vi "Dresden R2R Sputter 03.02.2018 IY24.vi"() -> ()   [LabVIEW 2009] (continued)
                                }
                                }
                                n29134 = local read "Semi"() -> (w34103:bool)
                                n29135 = Or(x=w34104, y=w34103) -> (x .or. y?=w34099:bool)
                                }
                                }
                                frame #4 {
                                n29136 = local read "Semi"() -> (w34113:bool)
                                n29137 = case shown="False" w34113 {
                                frame #0 {
                                n29138 = while {
                                i -> [w34119]
                                stop <- w34116 stop-if-true
                                n29139 = Greater?(x=w34119, y=50) -> (0:w34118:bool)
                                n29140 = case shown="True" w34118 {
                                frame #0 {
                                }
                                frame #1 {
                                n29141 = local write "Error Message"("" ("Error Message")) -> ()
                                n29142 = local write "Semi"(TRUE ("Semi")) -> ()
                                }
                                }
                                n29143 = local read "Casette_servo_start/stop_di"() -> (w34115:bool)
                                n29144 = case shown="True" w34115 {
                                tunnel: [TRUE FALSE] -> w34114
                                frame #0 {
                                }
                                frame #1 {
                                n29145 = local write "Casette_servo_start/stop_do"(FALSE ("Casette_servo_left_direction_do")) -> ()
                                n29146 = Wait Until Next ms Multiple(millisecond multiple=u32 500) -> ()  [unwired: 1 out]
                                }
                                }
                                n29147 = local read "Semi"() -> (w34117:bool)
                                n29148 = Or(x=w34114, y=w34117) -> (x .or. y?=w34116:bool)
                                }
                                }
                                frame #1 {
                                }
                                }
                                }
                                frame #5 {
                                n29149 = local read "Semi"() -> (w34127:bool)
                                n29150 = case shown="False" w34127 {
                                frame #0 {
                                n29151 = Wait (ms)(milliseconds to wait=u32 5000 ("millisecond multiple 8")) -> ()  [unwired: 1 out]
                                }
                                frame #1 {
                                }
                                }
                                }
                                frame #6 {
                                n29152 = local read "Semi"() -> (w34129:bool)
                                n29153 = case shown="False" w34129 {
                                frame #0 {
                                n29154 = while {
                                i -> [w34135]
                                stop <- w34132 stop-if-true
                                n29155 = Greater?(x=w34135, y=50) -> (0:w34134:bool)
                                n29156 = case shown="True" w34134 {
                                frame #0 {
                                }
                                frame #1 {
                                n29157 = local write "Error Message"("" ("Error Message")) -> ()
                                n29158 = local write "Semi"(TRUE ("Semi")) -> ()
                                }
                                }
                                n29159 = local read "Casette_servo_start/stop_di"() -> (w34131:bool)
                                n29160 = case shown="False" w34131 {
                                tunnel: [FALSE TRUE] -> w34130
                                frame #0 {
                                n29161 = local write "Casette_servo_start/stop_do"(TRUE ("Casette_servo_left_direction_do")) -> ()
                                n29162 = Wait Until Next ms Multiple(millisecond multiple=u32 500) -> ()  [unwired: 1 out]
                                }
                                frame #1 {
                                }
                                }
                                n29163 = local read "Semi"() -> (w34133:bool)
                                n29164 = Or(x=w34130, y=w34133) -> (x .or. y?=w34132:bool)
                                }
                                }
                                frame #1 {
                                }
                                }
                                }
                                frame #7 {
                                n29165 = local read "Semi"() -> (w34143:bool)
                                n29166 = case shown="False" w34143 {
                                frame #0 {
                                n29167 = while {
                                i -> [w34149]
                                stop <- w34146 stop-if-true
                                n29168 = Greater?(x=w34149, y=50) -> (0:w34148:bool)
                                n29169 = case shown="True" w34148 {
                                frame #0 {
                                }
                                frame #1 {
                                n29170 = local write "Error Message"("" ("Error Message")) -> ()
                                n29171 = local write "Semi"(TRUE ("Semi")) -> ()
                                }
                                }
                                n29172 = local read "Casette_servo_left_direction_di"() -> (w34145:bool)
                                n29173 = case shown="True" w34145 {
                                tunnel: [TRUE FALSE] -> w34144
                                frame #0 {
                                }
                                frame #1 {
                                n29174 = local write "Casette_servo_left_direction_do"(FALSE ("Casette_servo_left_direction_do")) -> ()
                                n29175 = Wait Until Next ms Multiple(millisecond multiple=u32 200) -> ()  [unwired: 1 out]
                                }
                                }
                                n29176 = local read "Semi"() -> (w34147:bool)
                                n29177 = Or(x=w34144, y=w34147) -> (x .or. y?=w34146:bool)
                                }
                                }
                                frame #1 {
                                }
                                }
                                }
                                frame #8 {
                                # "casette motion"
                                n29178 = while {
                                i -> [w34160]
                                stop <- w34157 stop-if-true
                                n29179 = Greater?(x=w34160, y=200) -> (0:w34161:bool)
                                n29180 = case shown="True" w34161 {
                                frame #0 {
                                }
                                frame #1 {
                                n29181 = local write "Semi"(TRUE ("Semi")) -> ()
                                }
                                }
                                n29182 = local read "Counter_read_data"() -> (w34165:i16)
                                n29183 = Less?(x=w34165, y=i16 0) -> (x < y?=w34164:bool)
                                n29184 = case shown="True" w34164 {
                                tunnel: [TRUE TRUE] -> w34163
                                frame #0 {
                                }
                                frame #1 {
                                n29185 = local write "Casette_servo_start/stop_do"(FALSE ("Casette_servo_start/stop_do")) -> ()
                                n29186 = Wait Until Next ms Multiple(millisecond multiple=u32 200) -> ()  [unwired: 1 out]
                                }
                                }
                                n29187 = local read "Semi"() -> (w34162:bool)
                                n29188 = Or(x=w34163, y=w34162) -> (x .or. y?=w34157:bool)
                                }
                                }
                                frame #9 {
                                n29189 = local read "Semi"() -> (w34171:bool)
                                n29190 = case shown="False" w34171 {
                                frame #0 {
                                n29191 = while {
                                i -> [w34177]
                                stop <- w34174 stop-if-true
                                n29192 = Greater?(x=w34177, y=50) -> (0:w34176:bool)
                                n29193 = case shown="True" w34176 {
                                frame #0 {
                                }
                                frame #1 {
                                n29194 = local write "Error Message"("" ("Error Message")) -> ()
                                n29195 = local write "Semi"(TRUE ("Semi")) -> ()
                                }
                                }
                                n29196 = local read "Casette_servo_start/stop_di"() -> (w34173:bool)
                                n29197 = case shown="True" w34173 {
                                tunnel: [TRUE FALSE] -> w34172
                                frame #0 {
                                }
                                frame #1 {
                                n29198 = local write "Casette_servo_start/stop_do"(FALSE ("Casette_servo_left_direction_do")) -> ()
                                n29199 = Wait Until Next ms Multiple(millisecond multiple=u32 500) -> ()  [unwired: 1 out]
                                }
                                }
                                n29200 = local read "Semi"() -> (w34175:bool)
                                n29201 = Or(x=w34172, y=w34175) -> (x .or. y?=w34174:bool)
                                }
                                }
                                frame #1 {
                                }
                                }
                                }
                                frame #10 {
                                n29202 = local read "Semi"() -> (w34185:bool)
                                n29203 = case shown="False" w34185 {
                                frame #0 {
                                n29204 = local write "SDC1 21b"(TRUE ("SDC1 21b")) -> ()
                                }
                                frame #1 {
                                }
                                }
                                }
                                }
                                }
                                frame #1 {
                                }
                                }
                                }
                                frame #1 {
                                }
                                }
                                }
                                }
                                }
                                frame #1 {
                                }
                                }
                                }
                                frame #1 {
                                n29205 = local read "Semi"() -> (w34187:bool)
                                n29206 = case shown="False" w34187 {
                                frame #0 {
                                n29207 = Wait (ms)(milliseconds to wait=u32 1000) -> ()  [unwired: 1 out]
                                n29208 = local write "SDC1 21"(TRUE ("SDC1 21")) -> ()
                                }
                                frame #1 {
                                }
                                }
                                }
                                }
                                }
                                frame #18 {
                                # "tm parameter"
                                n29209 = local read "Semi"() -> (w34190:bool)
                                n29210 = case shown="False" w34190 {
                                frame #0 {
                                n29211 = local read "Thickness_Monitor_Active"() -> (w34191:bool)
                                n29212 = case shown="True" w34191 {
                                frame #0 {
                                }
                                frame #1 {
                                n29213 = local read "Semi"() -> (w34192:bool)
                                n29214 = case shown="False" w34192 {
                                frame #0 {
                                n29215 = stacked-sequence {
                                frame #0 {
                                n29216 = local read "Semi"() -> (w34193:bool)
                                n29217 = case shown="False" w34193 {
                                frame #0 {
                                n29218 = local read "R Toooling_factor"() -> (w34194:dbl)
                                n29219 = local read "R Material_density"() -> (w34196:dbl)
                                n29220 = local read "R Z_factor"() -> (w34195:dbl)
                                n29221 = local write "Tooling_factor3"(w34194) -> ()
                                n29222 = local write "Material_density 3"(w34196) -> ()
                                n29223 = local write "Z_factor3"(w34195) -> ()
                                }
                                frame #1 {
                                }
                                }
                                }
                                frame #1 {
                                n29224 = local read "Semi"() -> (w34197:bool)
                                n29225 = case shown="False" w34197 {
                                frame #0 {
                                n29226 = Wait (ms)(milliseconds to wait=u32 1000) -> ()  [unwired: 1 out]
                                }
                                frame #1 {
                                }
                                }
                                }
                                frame #2 {
                                n29227 = local read "Semi"() -> (w34199:bool)
                                n29228 = case shown="False" w34199 {
                                frame #0 {
                                n29229 = local read "R Single RF Target material"() -> (w34200:string)
                                n29230 = Write to Text File(file (use dialog)=path path "D/VK-1701 System Files/Material Data/data3.txt", text=w34200) -> ()  [unwired: 2 in, 3 out]
                                }
                                frame #1 {
                                }
                                }
                                }
                                frame #3 {
                                n29231 = local read "Semi"() -> (w34202:bool)
                                n29232 = case shown="False" w34202 {
                                frame #0 {
                                n29233 = local write "SDC1 22"(TRUE ("SDC1 22")) -> ()
                                n29234 = Wait (ms)(milliseconds to wait=u32 1000) -> ()  [unwired: 1 out]
                                }
                                frame #1 {
                                }
                                }
                                }
                                }
                                }
                                frame #1 {
                                }
                                }
                                }
                                }
                                }
                                frame #1 {
                                }
                                }
                                }
                                frame #19 {
                                n29235 = local read "Semi"() -> (w34205:bool)
                                n29236 = case shown="False" w34205 {
                                frame #0 {
                                n29237 = local read "R_Web_selection"() -> (w34206:enum32{"Web", "Other"})
                                n29238 = case shown="\"Other\"" w34206 {
                                frame #0 {
                                }
                                frame #1 {
                                n29239 = local read "R_Thickness Selection"() -> (w34207:enum32{"Thickness", "Time"})
                                n29240 = case shown="\"Time\"" w34207 {
                                frame #0 {
                                n29241 = local read "Semi"() -> (w34210:bool)
                                n29242 = case shown="False" w34210 {
                                frame #0 {
                                n29243 = stacked-sequence {
                                frame #0 {
                                n29244 = local read "Semi"() -> (w34211:bool)
                                n29245 = case shown="False" w34211 {
                                frame #0 {
                                n29246 = local write "Tm3_auto_set_zero"(TRUE ("Tm1_auto_set_zero")) -> ()
                                n29247 = Wait (ms)(milliseconds to wait=u32 3000) -> ()  [unwired: 1 out]
                                }
                                frame #1 {
                                }
                                }
                                }
                                frame #1 {
                                n29248 = local read "Semi"() -> (w34214:bool)
                                n29249 = case shown="False" w34214 {
                                frame #0 {
                                n29250 = flat-sequence {
                                frame #0 {
                                n29251 = local write "Process_sputter 3"(u8 0 ("Process_sputter")) -> ()
                                }
                                frame #1 {
                                n29252 = Wait (ms)(milliseconds to wait=u32 1000) -> ()  [unwired: 1 out]
                                }
                                }
                                }
                                frame #1 {
                                }
                                }
                                }
                                frame #2 {
                                n29253 = local read "Semi"() -> (w34217:bool)
                                n29254 = case shown="False" w34217 {
                                frame #0 {
                                n29255 = local write "Process_sputter 3"(u8 0 ("Process_sputter")) -> ()
                                n29256 = property on="Process_tab_sputter 3" class="TabCtl (strict)"("Visible"=TRUE) -> ()  [unwired: 2 in, 2 out]
                                }
                                frame #1 {
                                }
                                }
                                }
                                frame #3 {
                                n29257 = local read "Semi"() -> (w34220:bool)
                                n29258 = case shown="False" w34220 {
                                frame #0 {
                                n29259 = while {
                                stop <- w34225 stop-if-true
                                n29260 = local read "R_Target Thickness Value"() -> (w34223:dbl)
                                n29261 = local read "Thickness 3-1"() -> (w34222:dbl)
                                n29262 = local read "Tm1_fail"() -> (w34233:bool)
                                n29263 = case shown="True" w34233 {
                                tunnel: [FALSE TRUE] -> w34226
                                frame #0 {
                                }
                                frame #1 {
                                n29264 = local write "Error Message"("Sputtering Process cancelled.\nPlease check TM1 connections." ("Error Message")) -> ()
                                }
                                }
                                n29265 = Divide(x=w34222, y=w34223) -> (x/y=w34231:dbl)
                                n29266 = Multiply(x=w34231, y=100.0) -> (x*y=w34229:dbl)
                                n29267 = Greater Or Equal?(x=w34229, y=100.0) -> (x >= y?=w34228:bool)
                                n29268 = local write "Target Thickness Sputter 3"(w34223) -> ()
                                n29269 = local write "Thickness_total 3"(w34222) -> ()
                                n29270 = local read "Abort_sputter 3"() -> (w34221:bool)
                                n29271 = local write "Process_sputter 3"(w34229) -> ()
                                n29272 = Wait Until Next ms Multiple(millisecond multiple=u32 300) -> ()  [unwired: 1 out]
                                n29273 = local read "Semi"() -> (w34227:bool)
                                n29274 = Compound Arithmetic op=OR(w34227, w34228, w34221, w34226) -> (w34225:bool)
                                }
                                }
                                frame #1 {
                                }
                                }
                                }
                                frame #4 {
                                n29275 = local read "Semi"() -> (w34237:bool)
                                n29276 = case shown="False" w34237 {
                                frame #0 {
                                w34238 = FALSE ("Abort_sputter")
                                n29277 = local write "Abort_sputter 3"(w34238) -> ()
                                n29278 = property on="Process_tab_sputter 3" class="TabCtl (strict)"("Visible"=w34238) -> ()  [unwired: 2 in, 2 out]
                                }
                                frame #1 {
                                }
                                }
                                }
                                frame #5 {
                                n29279 = local read "Tm1_fail"() -> (w34239:bool)
                                n29280 = case shown="False" w34239 {
                                frame #0 {
                                n29281 = Wait (ms)(milliseconds to wait=u32 1000) -> ()  [unwired: 1 out]
                                n29282 = local write "SDC1 23"(TRUE ("SDC1 23")) -> ()
                                }
                                frame #1 {
                                }
                                }
                                }
                                }
                                }
                                frame #1 {
                                }
                                }
                                }
                                frame #1 {
                                n29283 = local read "Semi"() -> (w34242:bool)
                                n29284 = case shown="False" w34242 {
                                frame #0 {
                                n29285 = stacked-sequence {
                                frame #0 {
                                n29286 = local read "Semi"() -> (w34243:bool)
                                n29287 = case shown="False" w34243 {
                                frame #0 {
                                w34244 = TRUE ("Tm1_auto_set_zero")
                                n29288 = local write "Tm3_auto_set_zero"(w34244) -> ()
                                n29289 = property on="Sputter_tab 3" class="TabCtl (strict)"("Visible"=w34244) -> ()  [unwired: 2 in, 2 out]
                                n29290 = Wait (ms)(milliseconds to wait=u32 1000) -> ()  [unwired: 1 out]
                                }
                                frame #1 {
                                }
                                }
                                }
                                frame #1 {
                                n29291 = local read "Semi"() -> (w34246:bool)
                                n29292 = case shown="False" w34246 {
                                frame #0 {
                                n29293 = while {
                                i -> [w34255]
                                stop <- w34254 stop-if-true
                                n29294 = Wait Until Next ms Multiple(millisecond multiple=u32 1000) -> ()  [unwired: 1 out]
                                n29295 = local read "R_Duration"() -> (w34256:dbl)
                                n29296 = local read "Sputter_cancel 3"() -> (w34247:bool)
                                n29297 = local read "Semi"() -> (w34251:bool)
                                n29298 = Multiply(x=w34256, y=60.0) -> (x*y=w34253:dbl)
                                n29299 = Greater?(x=w34255, y=w34253) -> (0:w34252:bool)
                                n29300 = Compound Arithmetic op=OR(w34251, w34247, w34252) -> (w34250:bool)
                                n29301 = local read "R_Duration"() -> (w34248:dbl)
                                n29302 = case shown="False" w34250 {
                                tunnel: w34255 -> [w34260 _]
                                tunnel: [FALSE TRUE] -> w34254
                                tunnel: w34253 -> [w34261 _]
                                frame #0 {
                                n29303 = Subtract(x=w34261, y=w34260) -> (x-y=w34258:dbl)
                                n29304 = local write "Sputter_left_time 3"(w34258) -> ()
                                }
                                frame #1 {
                                n29305 = property on="Sputter_tab 3" class="TabCtl (strict)"("Visible"=FALSE) -> ()  [unwired: 2 in, 2 out]
                                }
                                }
                                n29306 = local write "Sputter_set_time 3"(w34248) -> ()
                                }
                                }
                                frame #1 {
                                }
                                }
                                }
                                frame #2 {
                                n29307 = local write "Sputter_cancel 3"(FALSE ("Sputter_cancel")) -> ()
                                }
                                frame #3 {
                                n29308 = local write "SDC1 24"(TRUE ("SDC1 24")) -> ()
                                n29309 = Wait (ms)(milliseconds to wait=u32 1000) -> ()  [unwired: 1 out]
                                }
                                }
                                }
                                frame #1 {
                                }
                                }
                                }
                                }
                                n29310 = local read "Substrate Material"() -> (w34208:string)
                                n29311 = Write to Text File(file (use dialog)=path path "D/VK-1701 System Files/Material Data/data2.txt", text=w34208) -> ()  [unwired: 2 in, 3 out]
                                }
                                }
                                }
                                frame #1 {
                                }
                                }
                                }
                                frame #20 {
                                # "CLOSE DC"
                                n29312 = local read "Semi"() -> (w34267:bool)
                                n29313 = case shown="False" w34267 {
                                frame #0 {
                                n29314 = stacked-sequence {
                                frame #0 {
                                n29315 = local read "Semi"() -> (w34268:bool)
                                n29316 = case shown="False" w34268 {
                                frame #0 {
                                n29317 = local write "RF_auto_off"(TRUE ("Dc_auto_off")) -> ()
                                }
                                frame #1 {
                                }
                                }
                                }
                                frame #1 {
                                n29318 = local read "Semi"() -> (w34270:bool)
                                n29319 = case shown="False" w34270 {
                                frame #0 {
                                n29320 = Wait (ms)(milliseconds to wait=u32 1000) -> ()  [unwired: 1 out]
                                }
                                frame #1 {
                                }
                                }
                                }
                                frame #2 {
                                n29321 = local read "Semi"() -> (w34272:bool)
                                n29322 = case shown="False" w34272 {
                                frame #0 {
                                n29323 = local write "RF_forward_power_1"(0.0 ("Set DC Power :")) -> ()
                                }
                                frame #1 {
                                }
                                }
                                }
                                frame #3 {
                                n29324 = local read "Semi"() -> (w34274:bool)
                                n29325 = case shown="False" w34274 {
                                frame #0 {
                                n29326 = Wait (ms)(milliseconds to wait=u32 1000) -> ()  [unwired: 1 out]
                                }
                                frame #1 {
                                }
                                }
                                }
                                frame #4 {
                                n29327 = local read "Semi"() -> (w34276:bool)
                                n29328 = case shown="False" w34276 {
                                frame #0 {
                                n29329 = local write "RF set auto"(TRUE ("Dc_auto_set")) -> ()
                                }
                                frame #1 {
                                }
                                }
                                }
                                frame #5 {
                                n29330 = local read "Semi"() -> (w34278:bool)
                                n29331 = case shown="False" w34278 {
                                frame #0 {
                                n29332 = Wait (ms)(milliseconds to wait=u32 1000) -> ()  [unwired: 1 out]
                                }
                                frame #1 {
                                }
                                }
                                }
                                frame #6 {
                                n29333 = local read "Semi"() -> (w34280:bool)
                                n29334 = case shown="False" w34280 {
                                frame #0 {
                                n29335 = while {
                                i -> [w34288]
                                stop <- w34282 stop-if-true
                                n29336 = Greater?(x=w34288, y=600) -> (0:w34287:bool)
                                n29337 = case shown="True" w34287 {
                                frame #0 {
                                }
                                frame #1 {
                                n29338 = local write "Semi"(TRUE ("Semi")) -> ()
                                n29339 = local write "Error Message"("Sputter Process cancelled.\nPlease Check DC connections." ("Error Message")) -> ()
                                }
                                }
                                n29340 = local read "RF Net Power :"() -> (w34285:u32)
                                n29341 = Less?(x=w34285, y=10.0) -> (x < y?=w34281:bool)
                                n29342 = local read "Semi"() -> (w34283:bool)
                                n29343 = Wait Until Next ms Multiple(millisecond multiple=u32 500) -> ()  [unwired: 1 out]
                                n29344 = Compound Arithmetic op=OR(w34281, w34283) -> (w34282:bool)
                                }
                                }
                                frame #1 {
                                }
                                }
                                }
                                frame #7 {
                                n29345 = local read "Semi"() -> (w34292:bool)
                                n29346 = case shown="False" w34292 {
                                frame #0 {
                                n29347 = Wait (ms)(milliseconds to wait=u32 1000) -> ()  [unwired: 1 out]
                                n29348 = local write "SDC1 25"(TRUE ("SDC1 25")) -> ()
                                }
                                frame #1 {
                                }
                                }
                                }
                                }
                                }
                                frame #1 {
                                }
                                }
                                }
                                frame #21 {
                                # "PC-BV OPEN"
                                n29349 = stacked-sequence {
                                frame #0 {
                                n29350 = local read "Semi"() -> (w34295:bool)
                                n29351 = case shown="False" w34295 {
                                frame #0 {
                                n29352 = stacked-sequence {
                                frame #0 {
                                n29353 = local read "Semi"() -> (w34296:bool)
                                n29354 = case shown="False" w34296 {
                                frame #0 {
                                n29355 = local write "Pc_bv4_auto_open"(TRUE ("Tp1_auto_start")) -> ()
                                }
                                frame #1 {
                                }
                                }
                                }
                                frame #1 {
                                n29356 = local read "Semi"() -> (w34298:bool)
                                n29357 = case shown="False" w34298 {
                                frame #0 {
                                n29358 = Wait (ms)(milliseconds to wait=u32 1000) -> ()  [unwired: 1 out]
                                }
                                frame #1 {
                                }
                                }
                                }
                                frame #2 {
                                n29359 = local read "Semi"() -> (w34300:bool)
                                n29360 = case shown="False" w34300 {
                                frame #0 {
                                n29361 = while {
                                i -> [w34306]
                                stop <- w34302 stop-if-true
                                n29362 = local read "Pc_bv_opened_ch4"() -> (w34304:bool)
                                n29363 = Greater?(x=w34306, y=120) -> (0:w34305:bool)
                                n29364 = local read "Semi"() -> (w34303:bool)
                                n29365 = Compound Arithmetic op=OR(w34303, w34304, w34305) -> (w34302:bool)
                                n29366 = Wait (ms)(milliseconds to wait=u32 500) -> ()  [unwired: 1 out]
                                }
                                }
                                frame #1 {
                                }
                                }
                                }
                                frame #3 {
                                n29367 = local read "Semi"() -> (w34308:bool)
                                n29368 = case shown="False" w34308 {
                                frame #0 {
                                n29369 = local read "Pc_bv_opened_ch4"() -> (w34309:bool)
                                n29370 = case shown="False" w34309 {
                                frame #0 {
                                n29371 = local write "Pc_bv4_auto_open"(TRUE ("Pc_bv1_auto_open")) -> ()
                                }
                                frame #1 {
                                }
                                }
                                }
                                frame #1 {
                                }
                                }
                                }
                                frame #4 {
                                n29372 = local read "Semi"() -> (w34311:bool)
                                n29373 = case shown="False" w34311 {
                                frame #0 {
                                n29374 = local read "Pc_bv_opened_ch4"() -> (w34312:bool)
                                n29375 = case shown="False" w34312 {
                                frame #0 {
                                n29376 = Wait (ms)(milliseconds to wait=u32 1000) -> ()  [unwired: 1 out]
                                }
                                frame #1 {
                                }
                                }
                                }
                                frame #1 {
                                }
                                }
                                }
                                frame #5 {
                                n29377 = local read "Semi"() -> (w34314:bool)
                                n29378 = case shown="False" w34314 {
                                frame #0 {
                                n29379 = while {
                                i -> [w34320]
                                stop <- w34316 stop-if-true
                                n29380 = local read "Pc_bv_opened_ch4"() -> (w34318:bool)
                                n29381 = Greater?(x=w34320, y=120) -> (0:w34319:bool)
                                n29382 = local read "Semi"() -> (w34317:bool)
                                n29383 = Compound Arithmetic op=OR(w34317, w34318, w34319) -> (w34316:bool)
                                n29384 = Wait (ms)(milliseconds to wait=u32 500) -> ()  [unwired: 1 out]
                                }
                                }
                                frame #1 {
                                }
                                }
                                }
                                frame #6 {
                                n29385 = local read "Semi"() -> (w34322:bool)
                                n29386 = case shown="False" w34322 {
                                frame #0 {
                                n29387 = local read "Pc_bv_opened_ch4"() -> (w34323:bool)
                                n29388 = case shown="False" w34323 {
                                frame #0 {
                                n29389 = local write "Error Message"("Start up process  cancelled\nbecause  PC-BV not opened.\nPlease check PC-BV1 connections." ("Error Message")) -> ()
                                n29390 = Wait (ms)(milliseconds to wait=u32 1000) -> ()  [unwired: 1 out]
                                }
                                frame #1 {
                                }
                                }
                                }
                                frame #1 {
                                }
                                }
                                }
                                }
                                }
                                frame #1 {
                                }
                                }
                                }
                                frame #1 {
                                n29391 = local read "Semi"() -> (w34326:bool)
                                n29392 = case shown="False" w34326 {
                                frame #0 {
                                n29393 = Wait (ms)(milliseconds to wait=u32 1000) -> ()  [unwired: 1 out]
                                n29394 = local write "SDC1 28"(TRUE ("SDC1 28")) -> ()
                                }
                                frame #1 {
                                }
                                }
                                }
                                }
                                }
                                frame #22 {
                                # "set ar zero"
                                n29395 = stacked-sequence {
                                frame #0 {
                                n29396 = local read "Semi"() -> (w34329:bool)
                                n29397 = case shown="False" w34329 {
                                frame #0 {
                                n29398 = stacked-sequence {
                                frame #0 {
                                n29399 = local read "Semi"() -> (w34330:bool)
                                n29400 = case shown="False" w34330 {
                                frame #0 {
                                n29401 = local write "Ar_auto_set_zero_ch4"(TRUE ("Ar_auto_set_zero_ch1")) -> ()
                                }
                                frame #1 {
                                }
                                }
                                }
                                frame #1 {
                                n29402 = local read "Semi"() -> (w34332:bool)
                                n29403 = case shown="False" w34332 {
                                frame #0 {
                                n29404 = while {
                                i -> [w34335]
                                stop <- w34334 stop-if-true
                                n29405 = Greater?(x=w34335, y=150) -> (0:w34334:bool)
                                n29406 = local read "Semi"() -> (w34333:bool)
                                n29407 = case shown="False" w34333 {
                                tunnel: [FALSE TRUE] -> _
                                frame #0 {
                                n29408 = Wait Until Next ms Multiple(millisecond multiple=u32 200) -> ()  [unwired: 1 out]
                                }
                                frame #1 {
                                }
                                }
                                }
                                }
                                frame #1 {
                                }
                                }
                                }
                                frame #2 {
                                n29409 = local read "Semi"() -> (w34340:bool)
                                n29410 = case shown="False" w34340 {
                                frame #0 {
                                n29411 = local read "Ar_sccm_act 2"() -> (w34341:dbl)
                                n29412 = Less?(x=w34341, y=1) -> (x < y?=w34342:bool)
                                n29413 = case shown="False" w34342 {
                                frame #0 {
                                n29414 = local write "Ar_auto_set_zero_ch4"(TRUE ("Ar_auto_set_zero_ch1")) -> ()
                                }
                                frame #1 {
                                }
                                }
                                }
                                frame #1 {
                                }
                                }
                                }
                                frame #3 {
                                n29415 = local read "Semi"() -> (w34345:bool)
                                n29416 = case shown="False" w34345 {
                                frame #0 {
                                n29417 = local read "Ar_sccm_act 2"() -> (w34346:dbl)
                                n29418 = Less?(x=w34346, y=1) -> (x < y?=w34347:bool)
                                n29419 = case shown="False" w34347 {
                                frame #0 {
                                n29420 = while {
                                i -> [w34353]
                                stop <- w34350 stop-if-true
                                n29421 = Greater?(x=w34353, y=150) -> (0:w34351:bool)
                                n29422 = local read "Semi"() -> (w34349:bool)
                                n29423 = case shown="True" w34349 {
                                tunnel: [FALSE FALSE] -> w34352
                                frame #0 {
                                }
                                frame #1 {
                                n29424 = Wait Until Next ms Multiple(millisecond multiple=u32 200) -> ()  [unwired: 1 out]